vi "Dresden R2R Sputter 03.02.2018 IY24.vi"() -> ()   [LabVIEW 2009] (continued)
                      }
                    }
                  }
                }
              }
              frame #1 {
              }
            }
          }
          frame #17 {
            # "SET CASSETTE SERVO  SPEED 100"
            n12721 = local read "Semi"() -> (w19398:bool)
            n12722 = case shown="False" w19398 {
              frame #0 {
                n12723 = stacked-sequence {
                  frame #0 {
                    n12724 = while {
                      i -> [w19405]
                      stop <- w19401 stop-if-true
                      n12725 = local read "Ch3_Left_slow_di"() -> (w19399:bool)
                      n12726 = Greater?(x=w19405, y=1500) -> (0:w19404:bool)
                      n12727 = case shown="True" w19404 {
                        frame #0 {
                        }
                        frame #1 {
                          n12728 = local write "Semi"(TRUE ("Semi")) -> ()
                          n12729 = local write "Error Message"("Transfer process was cancelled.\nPlease check Casette & Sensor\nconnections." ("Error Message")) -> ()
                        }
                      }
                      n12730 = case shown="False" w19399 {
                        tunnel: [FALSE TRUE] -> w19402
                        frame #0 {
                          n12731 = Wait Until Next ms Multiple(millisecond multiple=u32 200) -> ()  [unwired: 1 out]
                        }
                        frame #1 {
                        }
                      }
                      n12732 = local read "Semi"() -> (w19400:bool)
                      n12733 = Or(x=w19402, y=w19400) -> (x .or. y?=w19401:bool)
                    }
                  }
                  frame #1 {
                    n12734 = disable-structure shown="Disabled" {
                      frame #0 {
                        n12735 = while {
                          i -> [w19420]
                          stop <- w19416 stop-if-true
                          n12736 = local read "Counter_read_data"() -> (w19413:i16)
                          n12737 = Greater?(x=w19420, y=5000) -> (0:w19419:bool)
                          n12738 = case shown="True" w19419 {
                            frame #0 {
                            }
                            frame #1 {
                              n12739 = local write "Semi"(TRUE ("Semi")) -> ()
                            }
                          }
                          n12740 = In Range and Coerce(upper limit=i16 1990, x=w19413, lower limit=i16 1980 ("upper limit")) -> (In Range?=w19411:bool)  [unwired: 1 out]
                          n12741 = case shown="True" w19411 {
                            tunnel: [FALSE TRUE] -> w19417
                            frame #0 {
                              n12742 = Wait Until Next ms Multiple(millisecond multiple=u32 200) -> ()  [unwired: 1 out]
                            }
                            frame #1 {
                            }
                          }
                          n12743 = local read "Semi"() -> (w19415:bool)
                          n12744 = Or(x=w19417, y=w19415) -> (x .or. y?=w19416:bool)
                        }
                      }
                      frame #1 {
                      }
                    }
                  }
                  frame #2 {
                    n12745 = local read "Semi"() -> (w19425:bool)
                    n12746 = case shown="False" w19425 {
                      frame #0 {
                        n12747 = local write "Cassette_servo_speed_value"(u16 100 ("Cassette_servo_speed_value")) -> ()
                      }
                      frame #1 {
                      }
                    }
                  }
                  frame #3 {
                    n12748 = local read "Semi"() -> (w19427:bool)
                    n12749 = case shown="False" w19427 {
                      frame #0 {
                        n12750 = Wait (ms)(milliseconds to wait=u32 200 ("millisecond multiple")) -> ()  [unwired: 1 out]
                      }
                      frame #1 {
                      }
                    }
                  }
                  frame #4 {
                    n12751 = local read "Semi"() -> (w19429:bool)
                    n12752 = case shown="False" w19429 {
                      frame #0 {
                        n12753 = local write "Cassette_servo_speed_auto_set"(TRUE ("Cassette_servo_speed_auto_set")) -> ()
                      }
                      frame #1 {
                      }
                    }
                  }
                  frame #5 {
                    n12754 = local read "Semi"() -> (w19431:bool)
                    n12755 = case shown="False" w19431 {
                      frame #0 {
                        n12756 = Wait (ms)(milliseconds to wait=u32 200 ("millisecond multiple")) -> ()  [unwired: 1 out]
                      }
                      frame #1 {
                      }
                    }
                  }
                  frame #6 {
                    n12757 = while {
                      i -> [w19436]
                      stop <- w19433 stop-if-true
                      n12758 = Greater?(x=w19436, y=50) -> (0:w19437:bool)
                      n12759 = local read "Cnt_Left_slow_di"() -> (w19439:bool)
                      n12760 = case shown="True" w19437 {
                        frame #0 {
                        }
                        frame #1 {
                          n12761 = local write "Semi"(TRUE ("Semi")) -> ()
                          n12762 = local write "Error Message"("\nPlease check connections." ("Error Message")) -> ()
                        }
                      }
                      n12763 = case shown="False" w19439 {
                        tunnel: [FALSE ("Cnt_Left_slow_do") TRUE ("Cnt_Left_slow_do")] -> w19435
                        frame #0 {
                          n12764 = Wait Until Next ms Multiple(millisecond multiple=u32 200) -> ()  [unwired: 1 out]
                          n12765 = local write "Cnt_Left_slow_do"(TRUE ("Cnt_Left_slow_do")) -> ()
                        }
                        frame #1 {
                        }
                      }
                      n12766 = local read "Semi"() -> (w19434:bool)
                      n12767 = Or(x=w19435, y=w19434) -> (x .or. y?=w19433:bool)
                    }
                  }
                  frame #7 {
                    n12768 = local read "Semi"() -> (w19446:bool)
                    n12769 = case shown="False" w19446 {
                      frame #0 {
                        n12770 = local write "CH1_2trns_12"(TRUE ("CH1_2trns_11")) -> ()
                        n12771 = Wait (ms)(milliseconds to wait=u32 500) -> ()  [unwired: 1 out]
                      }
                      frame #1 {
                      }
                    }
                  }
                }
              }
              frame #1 {
              }
            }
          }
          frame #18 {
            # "CASETTE STOP AND FIX"
            n12772 = local read "Semi"() -> (w19449:bool)
            n12773 = case shown="False" w19449 {
              frame #0 {
                n12774 = stacked-sequence {
                  frame #0 {
                    # "Center Casette stop"
                    n12775 = local read "Semi"() -> (w19450:bool)
                    n12776 = case shown="False" w19450 {
                      frame #0 {
                        n12777 = stacked-sequence {
                          frame #0 {
                            n12778 = while {
                              i -> [w19457]
                              stop <- w19452 stop-if-true
                              n12779 = local read "Ch3_Left_limit_di"() -> (w19451:bool)
                              n12780 = Greater?(x=w19457, y=600) -> (0:w19455:bool)
                              n12781 = case shown="True" w19455 {
                                frame #0 {
                                }
                                frame #1 {
                                n12782 = local write "Semi"(TRUE ("Semi")) -> ()
                                n12783 = local write "Error Message"("Transfer process was cancelled.\nPlease check Casette connections." ("Error Message")) -> ()
                                }
                              }
                              n12784 = case shown="False" w19451 {
                                tunnel: [FALSE TRUE] -> w19454
                                frame #0 {
                                n12785 = Wait Until Next ms Multiple(millisecond multiple=u32 200) -> ()  [unwired: 1 out]
                                }
                                frame #1 {
                                }
                              }
                              n12786 = local read "Semi"() -> (w19453:bool)
                              n12787 = Or(x=w19454, y=w19453) -> (x .or. y?=w19452:bool)
                            }
                          }
                          frame #1 {
                            n12788 = disable-structure shown="Disabled" {
                              frame #0 {
                                n12789 = while {
                                i -> [w19472]
                                stop <- w19467 stop-if-true
                                n12790 = local read "Counter_read_data"() -> (w19464:i16)
                                n12791 = Greater?(x=w19472, y=5000) -> (0:w19470:bool)
                                n12792 = case shown="True" w19470 {
                                frame #0 {
                                }
                                frame #1 {
                                n12793 = local write "Semi"(TRUE ("Semi")) -> ()
                                n12794 = local write "Error Message"("Transfer process was cancelled.\nPlease check Casette connections." ("Error Message")) -> ()
                                }
                                }
                                n12795 = In Range and Coerce(upper limit=i16 2209, x=w19464, lower limit=i16 2199 ("upper limit")) -> (In Range?=w19463:bool)  [unwired: 1 out]
                                n12796 = case shown="True" w19463 {
                                tunnel: [FALSE TRUE] -> w19469
                                frame #0 {
                                }
                                frame #1 {
                                n12797 = Wait Until Next ms Multiple(millisecond multiple=u32 500) -> ()  [unwired: 1 out]
                                }
                                }
                                n12798 = local read "Semi"() -> (w19468:bool)
                                n12799 = Or(x=w19469, y=w19468) -> (x .or. y?=w19467:bool)
                                }
                              }
                              frame #1 {
                              }
                            }
                          }
                          frame #2 {
                            n12800 = while {
                              i -> [w19484]
                              stop <- w19479 stop-if-true
                              n12801 = local read "Casette_servo_start/stop_di"() -> (w19478:bool)
                              n12802 = Greater?(x=w19484, y=50) -> (0:w19482:bool)
                              n12803 = case shown="True" w19482 {
                                frame #0 {
                                }
                                frame #1 {
                                n12804 = local write "Semi"(TRUE ("Semi")) -> ()
                                n12805 = local write "Error Message"("Transfer process was cancelled.\nPlease check Casette connections." ("Error Message")) -> ()
                                }
                              }
                              n12806 = case shown="True" w19478 {
                                tunnel: [TRUE FALSE] -> w19481
                                frame #0 {
                                }
                                frame #1 {
                                n12807 = Wait Until Next ms Multiple(millisecond multiple=u32 200) -> ()  [unwired: 1 out]
                                n12808 = local write "Casette_servo_start/stop_do"(FALSE ("Casette_servo_start/stop_di")) -> ()
                                }
                              }
                              n12809 = local read "Semi"() -> (w19480:bool)
                              n12810 = Or(x=w19481, y=w19480) -> (x .or. y?=w19479:bool)
                            }
                          }
                          frame #3 {
                            n12811 = local read "Semi"() -> (w19491:bool)
                            n12812 = case shown="False" w19491 {
                              frame #0 {
                                n12813 = Wait (ms)(milliseconds to wait=u32 200) -> ()  [unwired: 1 out]
                              }
                              frame #1 {
                              }
                            }
                          }
                          frame #4 {
                            n12814 = local read "Semi"() -> (w19493:bool)
                            n12815 = case shown="False" w19493 {
                              frame #0 {
                                n12816 = local write "Cassette_servo_speed_value"(u16 0 ("Cassette_servo_speed_value")) -> ()
                              }
                              frame #1 {
                              }
                            }
                          }
                          frame #5 {
                            n12817 = local read "Semi"() -> (w19495:bool)
                            n12818 = case shown="False" w19495 {
                              frame #0 {
                                n12819 = Wait (ms)(milliseconds to wait=u32 200) -> ()  [unwired: 1 out]
                              }
                              frame #1 {
                              }
                            }
                          }
                          frame #6 {
                            n12820 = local read "Semi"() -> (w19497:bool)
                            n12821 = case shown="False" w19497 {
                              frame #0 {
                                n12822 = local write "Cassette_servo_speed_auto_set"(TRUE ("Cassette_servo_speed_auto_set")) -> ()
                              }
                              frame #1 {
                              }
                            }
                          }
                          frame #7 {
                            n12823 = local read "Semi"() -> (w19499:bool)
                            n12824 = case shown="False" w19499 {
                              frame #0 {
                                n12825 = Wait (ms)(milliseconds to wait=u32 200) -> ()  [unwired: 1 out]
                              }
                              frame #1 {
                              }
                            }
                          }
                          frame #8 {
                            n12826 = local read "Semi"() -> (w19501:bool)
                            n12827 = case shown="False" w19501 {
                              frame #0 {
                                n12828 = local write "CH1_2trns_13"(TRUE ("CH1_2trns_9")) -> ()
                                n12829 = Wait (ms)(milliseconds to wait=u32 500) -> ()  [unwired: 1 out]
                              }
                              frame #1 {
                              }
                            }
                          }
                        }
                      }
                      frame #1 {
                      }
                    }
                  }
                  frame #1 {
                    # "CASETTE FIX DOWN CH2"
                    n12830 = local read "Semi"() -> (w19504:bool)
                    n12831 = case shown="False" w19504 {
                      frame #0 {
                        n12832 = stacked-sequence {
                          frame #0 {
                            n12833 = local read "Semi"() -> (w19505:bool)
                            n12834 = case shown="False" w19505 {
                              frame #0 {
                                n12835 = while {
                                i -> [w19512]
                                stop <- w19507 stop-if-true
                                n12836 = Greater?(x=w19512, y=50) -> (0:w19510:bool)
                                n12837 = local read "Ch3_Cst_fix_down_di"() -> (w19506:bool)
                                n12838 = case shown="True" w19510 {
                                frame #0 {
                                }
                                frame #1 {
                                n12839 = local write "Semi"(TRUE ("Semi")) -> ()
                                n12840 = local write "Error Message"("Up/Down positions could not reach\nthe down position.\nPlease check connections." ("Error Message")) -> ()
                                }
                                }
                                n12841 = case shown="False" w19506 {
                                tunnel: [FALSE TRUE] -> w19509
                                frame #0 {
                                n12842 = Wait Until Next ms Multiple(millisecond multiple=u32 200) -> ()  [unwired: 1 out]
                                n12843 = local write "Ch3_Cst_fix_do"(TRUE ("Ch1_pet_cool_up_do")) -> ()
                                }
                                frame #1 {
                                }
                                }
                                n12844 = local read "Semi"() -> (w19508:bool)
                                n12845 = Or(x=w19509, y=w19508) -> (x .or. y?=w19507:bool)
                                }
                              }
                              frame #1 {
                              }
                            }
                          }
                          frame #1 {
                            n12846 = local read "Semi"() -> (w19519:bool)
                            n12847 = case shown="False" w19519 {
                              frame #0 {
                                n12848 = local write "CH1_2trns_14"(TRUE ("CH1_2trns_9")) -> ()
                                n12849 = Wait (ms)(milliseconds to wait=u32 500) -> ()  [unwired: 1 out]
                              }
                              frame #1 {
                              }
                            }
                          }
                        }
                      }
                      frame #1 {
                      }
                    }
                  }
                  frame #2 {
                    n12850 = local read "Semi"() -> (w19522:bool)
                    n12851 = case shown="False" w19522 {
                      frame #0 {
                        n12852 = stacked-sequence {
                          frame #0 {
                            n12853 = local read "Semi"() -> (w19523:bool)
                            n12854 = case shown="False" w19523 {
                              frame #0 {
                                n12855 = while {
                                i -> [w19530]
                                stop <- w19525 stop-if-true
                                n12856 = Greater?(x=w19530, y=50) -> (0:w19528:bool)
                                n12857 = local read "Ch2_trns_gv_bp2_di"() -> (w19524:bool)
                                n12858 = case shown="True" w19528 {
                                frame #0 {
                                }
                                frame #1 {
                                n12859 = local write "Semi"(TRUE ("Semi")) -> ()
                                n12860 = local write "Error Message"("Transfer process was cancelled.\nPlease check CH1-Trns-GV connections." ("Error Message")) -> ()
                                }
                                }
                                n12861 = case shown="True" w19524 {
                                tunnel: [TRUE FALSE] -> w19527
                                frame #0 {
                                }
                                frame #1 {
                                n12862 = Wait Until Next ms Multiple(millisecond multiple=u32 200) -> ()  [unwired: 1 out]
                                n12863 = local write "Ch2_trns_gv_bp2_do"(FALSE ("Ch1_pet_cool_up_do")) -> ()
                                }
                                }
                                n12864 = local read "Semi"() -> (w19526:bool)
                                n12865 = Or(x=w19527, y=w19526) -> (x .or. y?=w19525:bool)
                                }
                              }
                              frame #1 {
                              }
                            }
                          }
                          frame #1 {
                            n12866 = local read "Semi"() -> (w19537:bool)
                            n12867 = case shown="False" w19537 {
                              frame #0 {
                                n12868 = Wait (ms)(milliseconds to wait=u32 500) -> ()  [unwired: 1 out]
                              }
                              frame #1 {
                              }
                            }
                          }
                          frame #2 {
                            n12869 = local read "Semi"() -> (w19539:bool)
                            n12870 = case shown="False" w19539 {
                              frame #0 {
                                n12871 = while {
                                i -> [w19546]
                                stop <- w19541 stop-if-true
                                n12872 = Greater?(x=w19546, y=50) -> (0:w19544:bool)
                                n12873 = local read "Ch3_Trns_gv_bp_di"() -> (w19540:bool)
                                n12874 = case shown="True" w19544 {
                                frame #0 {
                                }
                                frame #1 {
                                n12875 = local write "Semi"(TRUE ("Semi")) -> ()
                                n12876 = local write "Error Message"("Transfer process was cancelled.\nPlease check CH1-Trns-GV connections." ("Error Message")) -> ()
                                }
                                }
                                n12877 = case shown="True" w19540 {
                                tunnel: [TRUE FALSE] -> w19543
                                frame #0 {
                                }
                                frame #1 {
                                n12878 = local write "Ch3_Trns_gv_bp_do"(FALSE ("Ch1_pet_cool_up_do")) -> ()
                                n12879 = Wait Until Next ms Multiple(millisecond multiple=u32 200) -> ()  [unwired: 1 out]
                                }
                                }
                                n12880 = local read "Semi"() -> (w19542:bool)
                                n12881 = Or(x=w19543, y=w19542) -> (x .or. y?=w19541:bool)
                                }
                              }
                              frame #1 {
                              }
                            }
                          }
                          frame #3 {
                            n12882 = local read "Semi"() -> (w19553:bool)
                            n12883 = case shown="False" w19553 {
                              frame #0 {
                                n12884 = Wait (ms)(milliseconds to wait=u32 500) -> ()  [unwired: 1 out]
                              }
                              frame #1 {
                              }
                            }
                          }
                        }
                      }
                      frame #1 {
                      }
                    }
                  }
                  frame #3 {
                    n12885 = local read "Semi"() -> (w19555:bool)
                    n12886 = case shown="False" w19555 {
                      frame #0 {
                        n12887 = stacked-sequence {
                          frame #0 {
                            n12888 = local read "Semi"() -> (w19556:bool)
                            n12889 = case shown="False" w19556 {
                              frame #0 {
                                n12890 = local write "Ch2_Trns_gv_open_do"(FALSE ("Ch1_pet_cool_up_do")) -> ()
                              }
                              frame #1 {
                              }
                            }
                          }
                          frame #1 {
                            n12891 = local read "Semi"() -> (w19558:bool)
                            n12892 = case shown="False" w19558 {
                              frame #0 {
                                n12893 = while {
                                i -> [w19565]
                                stop <- w19560 stop-if-true
                                n12894 = Greater?(x=w19565, y=500) -> (0:w19563:bool)
                                n12895 = local read "Ch2_Trns_gv_close_di"() -> (w19559:bool)
                                n12896 = case shown="True" w19563 {
                                frame #0 {
                                }
                                frame #1 {
                                n12897 = local write "Semi"(TRUE ("Semi")) -> ()
                                n12898 = local write "Error Message"("Transfer process was cancelled.\nPlease check  GV connections." ("Error Message")) -> ()
                                }
                                }
                                n12899 = case shown="False" w19559 {
                                tunnel: [FALSE TRUE] -> w19562
                                frame #0 {
                                n12900 = Wait Until Next ms Multiple(millisecond multiple=u32 200) -> ()  [unwired: 1 out]
                                n12901 = local write "Ch2_Trns_gv_close_do"(TRUE ("Ch1_pet_cool_up_do")) -> ()
                                }
                                frame #1 {
                                }
                                }
                                n12902 = local read "Semi"() -> (w19561:bool)
                                n12903 = Or(x=w19562, y=w19561) -> (x .or. y?=w19560:bool)
                                }
                              }
                              frame #1 {
                              }
                            }
                          }
                          frame #2 {
                            n12904 = local read "Semi"() -> (w19572:bool)
                            n12905 = case shown="False" w19572 {
                              frame #0 {
                                n12906 = local write "CH1_2trns_17"(TRUE ("CH1_2trns_9")) -> ()
                                n12907 = Wait (ms)(milliseconds to wait=u32 500) -> ()  [unwired: 1 out]
                              }
                              frame #1 {
                              }
                            }
                          }
                        }
                      }
                      frame #1 {
                      }
                    }
                  }
                  frame #4 {
                    # "PET COOL DOWN OF CH2"
                    n12908 = local read "Semi"() -> (w19575:bool)
                    n12909 = case shown="False" w19575 {
                      frame #0 {
                        n12910 = stacked-sequence {
                          frame #0 {
                            n12911 = local read "Semi"() -> (w19576:bool)
                            n12912 = case shown="False" w19576 {
                              frame #0 {
                                n12913 = local write "Ch3_Pet_cool_up_do"(FALSE ("Ch1_pet_cool_up_do")) -> ()
                              }
                              frame #1 {
                              }
                            }
                          }
                          frame #1 {
                            n12914 = local read "Semi"() -> (w19578:bool)
                            n12915 = case shown="False" w19578 {
                              frame #0 {
                                n12916 = while {
                                i -> [w19585]
                                stop <- w19580 stop-if-true
                                n12917 = Greater?(x=w19585, y=300) -> (0:w19583:bool)
                                n12918 = case shown="True" w19583 {
                                frame #0 {
                                }
                                frame #1 {
                                n12919 = local write "Semi"(TRUE ("Semi")) -> ()
                                n12920 = local write "Error Message"("SBS Cool Up/Down positions could not reach\nthe down position.\nPlease check connections." ("Error Message")) -> ()
                                }
                                }
                                n12921 = local read "Ch3_Pet_cool_down_di"() -> (w19579:bool)
                                n12922 = case shown="False" w19579 {
                                tunnel: [FALSE TRUE] -> w19582
                                frame #0 {
                                n12923 = Wait Until Next ms Multiple(millisecond multiple=u32 200) -> ()  [unwired: 1 out]
                                n12924 = local write "Ch3_Pet_cool_down_do"(TRUE ("Ch1_pet_cool_up_do")) -> ()
                                }
                                frame #1 {
                                }
                                }
                                n12925 = local read "Semi"() -> (w19581:bool)
                                n12926 = Or(x=w19582, y=w19581) -> (x .or. y?=w19580:bool)
                                }
                              }
                              frame #1 {
                              }
                            }
                          }
                          frame #2 {
                            n12927 = local read "Semi"() -> (w19592:bool)
                            n12928 = case shown="False" w19592 {
                              frame #0 {
                                n12929 = local write "CH1_2trns_15"(TRUE ("CH1_2trns_9")) -> ()
                                n12930 = Wait (ms)(milliseconds to wait=u32 500) -> ()  [unwired: 1 out]
                              }
                              frame #1 {
                              }
                            }
                          }
                        }
                      }
                      frame #1 {
                      }
                    }
                  }
                  frame #5 {
                    # "SRV PIS FOR"
                    n12931 = local read "Semi"() -> (w19595:bool)
                    n12932 = case shown="False" w19595 {
                      frame #0 {
                        n12933 = stacked-sequence {
                          frame #0 {
                            n12934 = local read "Semi"() -> (w19596:bool)
                            n12935 = case shown="False" w19596 {
                              frame #0 {
                                n12936 = local write "Ch3_SRV1_PIST_Back_do"(FALSE ("Ch1_pet_cool_up_do")) -> ()
                              }
                              frame #1 {
                              }
                            }
                          }
                          frame #1 {
                            n12937 = local read "Semi"() -> (w19598:bool)
                            n12938 = case shown="False" w19598 {
                              frame #0 {
                                n12939 = while {
                                i -> [w19605]
                                stop <- w19600 stop-if-true
                                n12940 = Greater?(x=w19605, y=100) -> (0:w19603:bool)
                                n12941 = local read "Ch3_SRV1_PIST For_di"() -> (w19599:bool)
                                n12942 = case shown="True" w19603 {
                                frame #0 {
                                }
                                frame #1 {
                                n12943 = local write "Semi"(TRUE ("Semi")) -> ()
                                n12944 = local write "Error Message"("For/Back positions could not reach\nthe forward position.\nPlease check connections." ("Error Message")) -> ()
                                }
                                }
                                n12945 = case shown="False" w19599 {
                                tunnel: [FALSE TRUE] -> w19602
                                frame #0 {
                                n12946 = Wait Until Next ms Multiple(millisecond multiple=u32 200) -> ()  [unwired: 1 out]
                                n12947 = local write "Ch3_SRV1_PIST For_do"(TRUE ("Ch1_pet_cool_up_do")) -> ()
                                }
                                frame #1 {
                                }
                                }
                                n12948 = local read "Semi"() -> (w19601:bool)
                                n12949 = Or(x=w19602, y=w19601) -> (x .or. y?=w19600:bool)
                                }
                              }
                              frame #1 {
                              }
                            }
                          }
                          frame #2 {
                            n12950 = local read "Semi"() -> (w19612:bool)
                            n12951 = case shown="False" w19612 {
                              frame #0 {
                                n12952 = local write "CH1_2trns_16"(TRUE ("CH1_2trns_9")) -> ()
                                n12953 = Wait (ms)(milliseconds to wait=u32 500) -> ()  [unwired: 1 out]
                              }
                              frame #1 {
                              }
                            }
                          }
                        }
                      }
                      frame #1 {
                      }
                    }
                  }
                }
              }
              frame #1 {
              }
            }
          }
          frame #19 {
            # "Sensors deactive"
            n12954 = local read "Semi"() -> (w19615:bool)
            n12955 = case shown="False" w19615 {
              frame #0 {
                n12956 = stacked-sequence {
                  frame #0 {
                    n12957 = local read "Semi"() -> (w19616:bool)
                    n12958 = case shown="False" w19616 {
                      frame #0 {
                        n12959 = while {
                          i -> [w19619]
                          stop <- w19620 stop-if-true
                          n12960 = Greater?(x=w19619, y=50) -> (0:w19617:bool)
                          n12961 = local read "Cnt_Right_slow_di"() -> (w19623:bool)
                          n12962 = case shown="True" w19617 {
                            frame #0 {
                            }
                            frame #1 {
                              n12963 = local write "Semi"(TRUE ("Semi")) -> ()
                              n12964 = local write "Error Message"("Transfer process was\ncancelled.Please check right slow sensor." ("Error Message")) -> ()
                            }
                          }
                          n12965 = case shown="False" w19623 {
                            tunnel: [FALSE ("Ch1_pet_cool_up_do") TRUE ("Ch1_pet_cool_up_do")] -> w19622
                            frame #0 {
                              n12966 = Wait Until Next ms Multiple(millisecond multiple=u32 200) -> ()  [unwired: 1 out]
                              n12967 = local write "Cnt_Right_slow_do"(TRUE ("Ch1_pet_cool_up_do")) -> ()
                            }
                            frame #1 {
                            }
                          }
                          n12968 = local read "Semi"() -> (w19621:bool)
                          n12969 = Or(x=w19622, y=w19621) -> (x .or. y?=w19620:bool)
                        }
                      }
                      frame #1 {
                      }
                    }
                  }
                  frame #1 {
                    n12970 = local read "Semi"() -> (w19630:bool)
                    n12971 = case shown="False" w19630 {
                      frame #0 {
                        n12972 = while {
                          i -> [w19633]
                          stop <- w19634 stop-if-true
                          n12973 = Greater?(x=w19633, y=50) -> (0:w19631:bool)
                          n12974 = local read "Cnt_Right_limit_di"() -> (w19637:bool)
                          n12975 = case shown="True" w19631 {
                            frame #0 {
                            }
                            frame #1 {
                              n12976 = local write "Semi"(TRUE ("Semi")) -> ()
                              n12977 = local write "Error Message"("Transfer process was\ncancelled.Please check right limit sensor." ("Error Message")) -> ()
                            }
                          }
                          n12978 = case shown="False" w19637 {
                            tunnel: [FALSE ("Ch1_pet_cool_up_do") TRUE ("Ch1_pet_cool_up_do")] -> w19636
                            frame #0 {
                              n12979 = Wait Until Next ms Multiple(millisecond multiple=u32 200) -> ()  [unwired: 1 out]
                              n12980 = local write "Cnt_Right_limit_do"(TRUE ("Ch1_pet_cool_up_do")) -> ()
                            }
                            frame #1 {
                            }
                          }
                          n12981 = local read "Semi"() -> (w19635:bool)
                          n12982 = Or(x=w19636, y=w19635) -> (x .or. y?=w19634:bool)
                        }
                      }
                      frame #1 {
                      }
                    }
                  }
                  frame #2 {
                    n12983 = local read "Semi"() -> (w19644:bool)
                    n12984 = case shown="False" w19644 {
                      frame #0 {
                        n12985 = while {
                          i -> [w19647]
                          stop <- w19648 stop-if-true
                          n12986 = Greater?(x=w19647, y=50) -> (0:w19645:bool)
                          n12987 = local read "Cnt_Left_slow_di"() -> (w19651:bool)
                          n12988 = case shown="True" w19645 {
                            frame #0 {
                            }
                            frame #1 {
                              n12989 = local write "Semi"(TRUE ("Semi")) -> ()
                              n12990 = local write "Error Message"("Transfer process was\ncancelled.Please check left slow sensor." ("Error Message")) -> ()
                            }
                          }
                          n12991 = case shown="False" w19651 {
                            tunnel: [FALSE ("Ch1_pet_cool_up_do") TRUE ("Ch1_pet_cool_up_do")] -> w19650
                            frame #0 {
                              n12992 = Wait Until Next ms Multiple(millisecond multiple=u32 200) -> ()  [unwired: 1 out]
                              n12993 = local write "Cnt_Left_slow_do"(TRUE ("Ch1_pet_cool_up_do")) -> ()
                            }
                            frame #1 {
                            }
                          }
                          n12994 = local read "Semi"() -> (w19649:bool)
                          n12995 = Or(x=w19650, y=w19649) -> (x .or. y?=w19648:bool)
                        }
                      }
                      frame #1 {
                      }
                    }
                  }
                  frame #3 {
                    n12996 = local read "Semi"() -> (w19658:bool)
                    n12997 = case shown="False" w19658 {
                      frame #0 {
                        n12998 = while {
                          i -> [w19661]
                          stop <- w19662 stop-if-true
                          n12999 = Greater?(x=w19661, y=50) -> (0:w19659:bool)
                          n13000 = local read "Cnt_Left_limit_di"() -> (w19665:bool)
                          n13001 = case shown="True" w19659 {
                            frame #0 {
                            }
                            frame #1 {
                              n13002 = local write "Semi"(TRUE ("Semi")) -> ()
                              n13003 = local write "Error Message"("Transfer process was\ncancelled.Please check left limit sensor." ("Error Message")) -> ()
                            }
                          }
                          n13004 = case shown="False" w19665 {
                            tunnel: [FALSE ("Ch1_pet_cool_up_do") TRUE ("Ch1_pet_cool_up_do")] -> w19664
                            frame #0 {
                              n13005 = Wait Until Next ms Multiple(millisecond multiple=u32 200) -> ()  [unwired: 1 out]
                              n13006 = local write "Cnt_Left_limit_do"(TRUE ("Ch1_pet_cool_up_do")) -> ()
                            }
                            frame #1 {
                            }
                          }
                          n13007 = local read "Semi"() -> (w19663:bool)
                          n13008 = Or(x=w19664, y=w19663) -> (x .or. y?=w19662:bool)
                        }
                      }
                      frame #1 {
                      }
                    }
                  }
                  frame #4 {
                    n13009 = local read "Semi"() -> (w19672:bool)
                    n13010 = case shown="False" w19672 {
                      frame #0 {
                        n13011 = local write "CH1_2trns_18"(TRUE ("CH1_2trns_7")) -> ()
                        n13012 = Wait (ms)(milliseconds to wait=u32 500) -> ()  [unwired: 1 out]
                      }
                      frame #1 {
                      }
                    }
                  }
                }
              }
              frame #1 {
              }
            }
          }
          frame #20 {
            n13013 = local read "Semi"() -> (w19675:bool)
            n13014 = case shown="False" w19675 {
              frame #0 {
                n13015 = local write "CH1_2trns_19"(TRUE ("CH1_2trns_18")) -> ()
                n13016 = local write "Cnt_Do_Buzzer"(TRUE ("Transfer_ch1_2")) -> ()
                n13017 = Wait (ms)(milliseconds to wait=u32 1500) -> ()  [unwired: 1 out]
              }
              frame #1 {
              }
            }
          }
          frame #21 {
            n13018 = local read "Semi"() -> (w19679:bool)
            n13019 = case shown="False" w19679 {
              frame #0 {
                n13020 = local write "ch_present_position"(3.0 ("ch_present_position")) -> ()
                n13021 = local write "Transfer_ch2_3"(FALSE ("Transfer_ch1_2")) -> ()
                n13022 = local write "Cnt_Do_Buzzer"(FALSE ("Transfer_ch1_2")) -> ()
                n13023 = Wait (ms)(milliseconds to wait=u32 500) -> ()  [unwired: 1 out]
              }
              frame #1 {
              }
            }
          }
        }
      }
      frame #4 {
        n13024 = stacked-sequence {
          frame #0 {
            n13025 = Wait (ms)(milliseconds to wait=u32 1500) -> ()  [unwired: 1 out]
            n13026 = local write "Clean_trnsfr_3_2"(TRUE ("Clean_trnsfr_1_2")) -> ()
            n13027 = local write "system_status"("Chamber 3 to Chamber 2 Transfer Process in Progress." ("system_status")) -> ()
            n13028 = local write "final_process_messages"("Chamber 3 to Chamber 2  Transfer Process was completed." ("final_process_messages")) -> ()
          }
          frame #1 {
            n13029 = stacked-sequence {
              frame #0 {
                n13030 = local write "Routine_check_transfer"(TRUE ("Routine_check_transfer")) -> ()
                n13031 = Wait (ms)(milliseconds to wait=u32 100) -> ()  [unwired: 1 out]
              }
              frame #1 {
                n13032 = while {
                  i -> [w19697]
                  stop <- w19693 stop-if-true
                  n13033 = Greater Or Equal?(x=w19697, y=1500) -> (x >= y?=w19694:bool)
                  n13034 = Wait Until Next ms Multiple(millisecond multiple=u32 200) -> ()  [unwired: 1 out]
                  n13035 = case shown="True" w19694 {